vi "UHR-Fleezers Control (host) - 10.6.vi"() -> ()   [LabVIEW 2010] (continued)
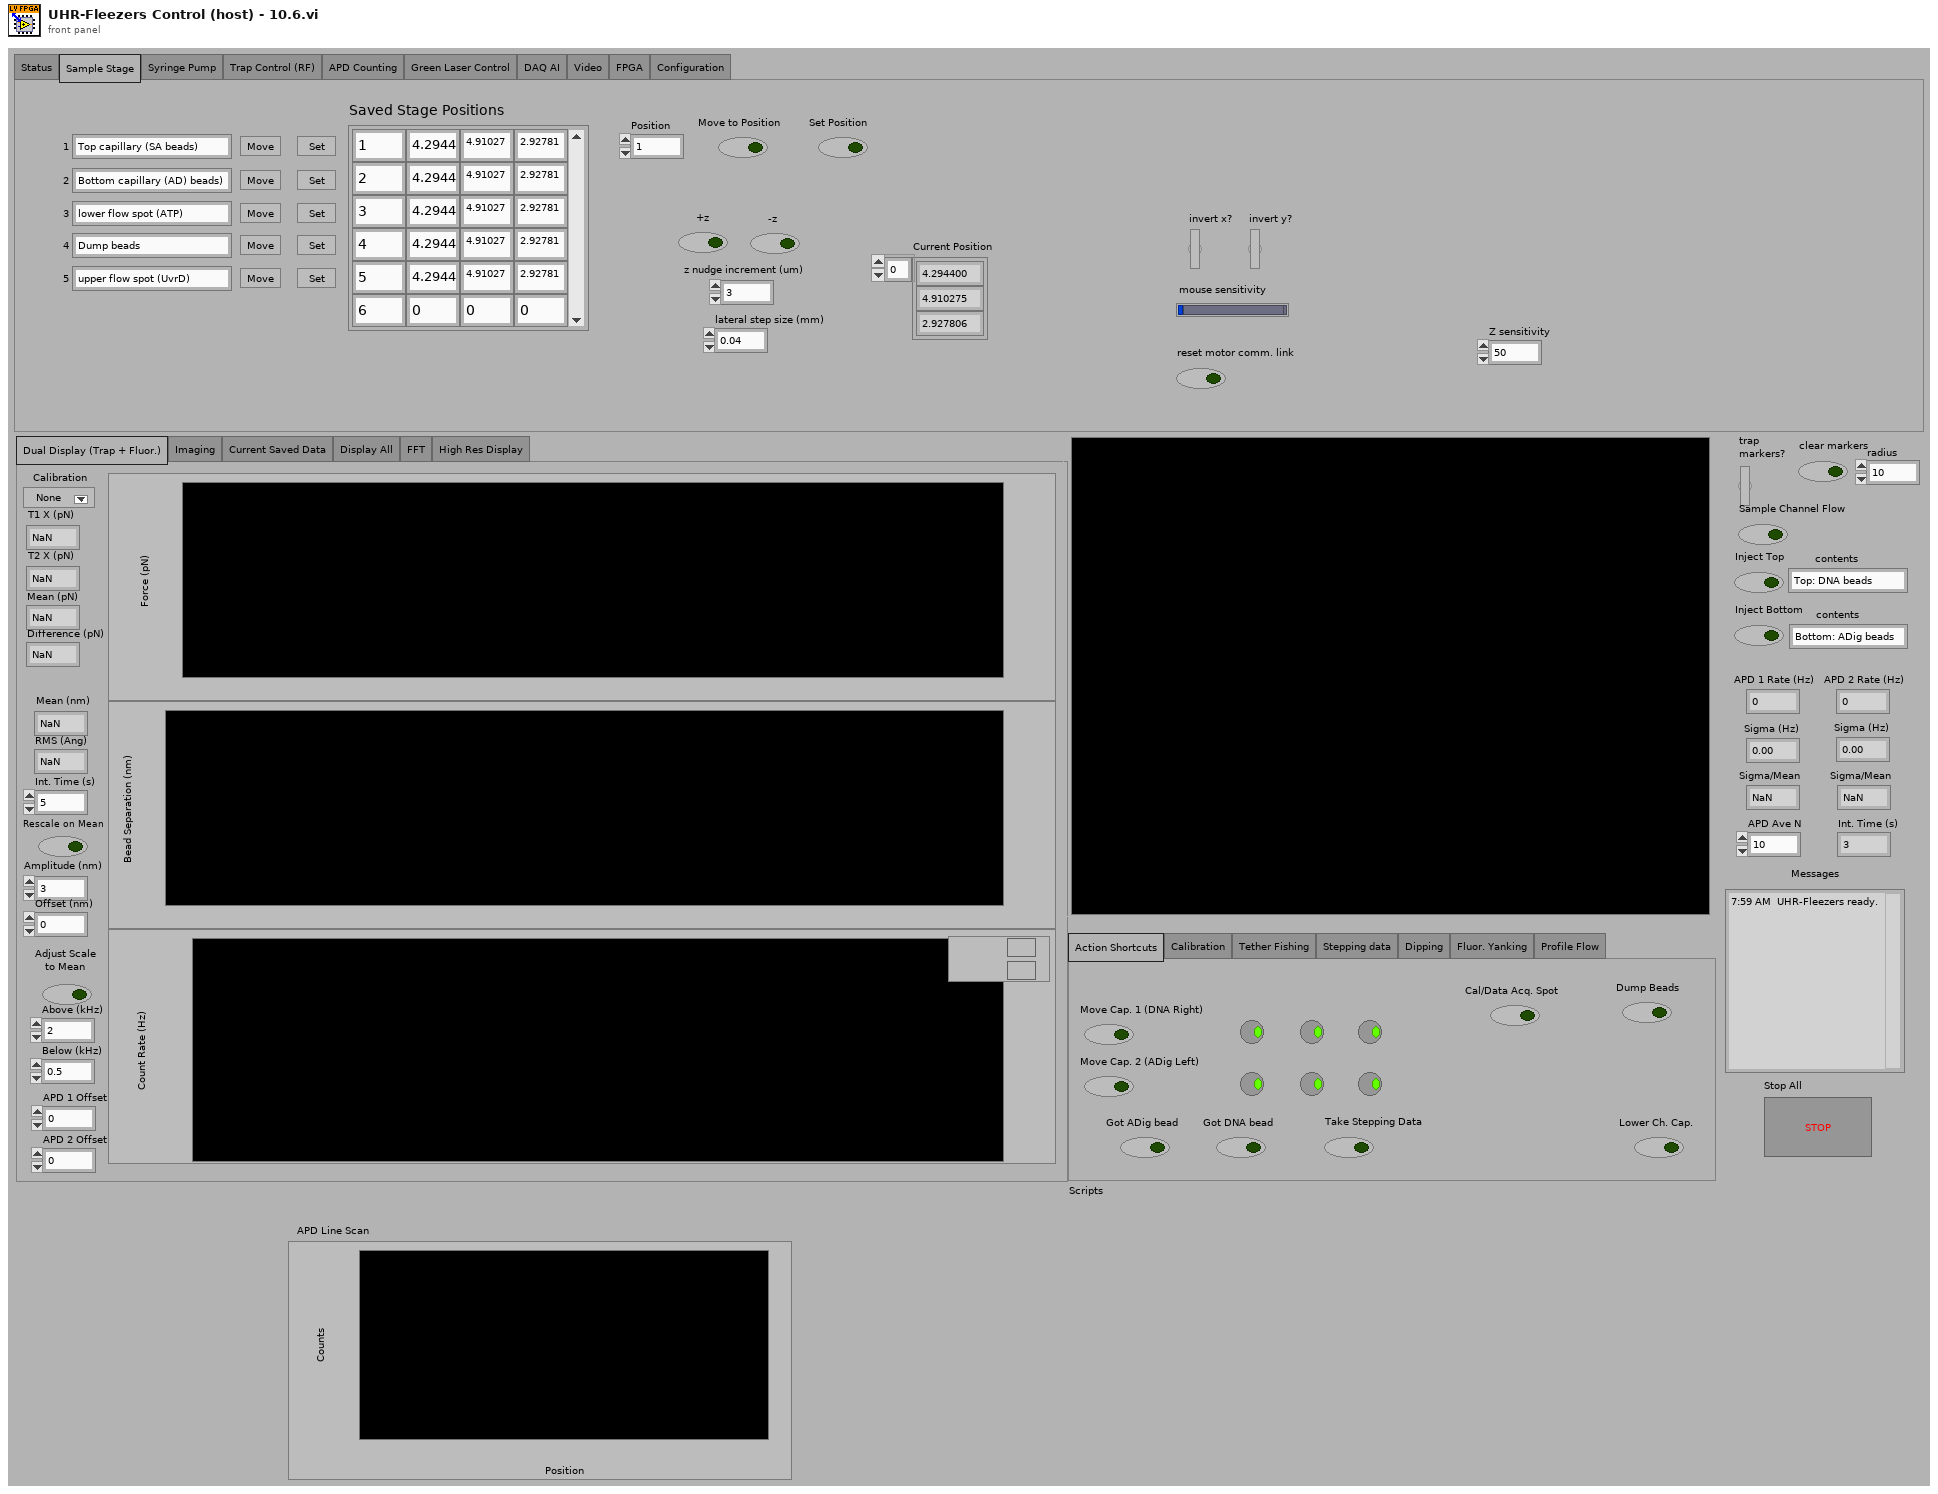
[diagram p1: front panel]
types:
  T1 = enum32{"Action Shortcuts", "Calibration", "Tether Fishing", "Stepping data", "Dipping", "Fluor. Yanking", "Profile Flow"}
  T2 = typedef "IMAQ Image.ctl" = refnum<image>
  T3 = enum32{"Dual Display (Trap + Fluor.)", "Imaging", "Current Saved Data", "Display All", "FFT", "High Res Display"}
  T4 = enum32{"Status", "Sample Stage", "Syringe Pump", "Trap Control (RF)", "APD Counting", "Green Laser Control", "DAQ AI", "Video", "FPGA", "Configuration"}
  T5 = cluster{"Pump 1":cluster{"Diameter (mm)":dbl, "Units":dbl, "Volume":dbl, "Rate":dbl}, "Pump 2":cluster{"Diameter (mm)":dbl, "Units":dbl, "Volume":dbl, "Rate":dbl}, "Pump 3":cluster{"Diameter (mm)":dbl, "Units":dbl, "Volume":dbl, "Rate":dbl}}
  T6 = enum32{"IR Laser Interlacing (Direct RF Board Control Method)", "AOD Raster Scan", "Feedback on Trap Intensity", "Feedback on Trap Position"}
  T7 = typedef "LVPoint32TypeDef.ctl" = cluster{"Horizontal":i32, "Vertical":i32}
  T8 = cluster{"Scan Range AOD (nm) 2":dbl, "Step Size AOD (nm) 2":dbl, "Scan Speed AOD (nm/s) 2":dbl, "Number of scans (AOD) 2":u16, "Label":string}[]
  T9 = cluster{"Set 1":cluster{"proportional gain (Kc)":i16, "integral gain (Kc*Ts/Ti)":i16, "derivative gain (Kc*Td/Ts)":i16}, "Set 2":cluster{"proportional gain (Kc)":i16, "integral gain (Kc*Ts/Ti)":i16, "derivative gain (Kc*Td/Ts)":i16}}
  T10 = cluster{"Trap 1":fxp<+/-,16,1>, "Trap 2":fxp<+/-,16,1>}
  T11 = cluster{"proportional gain (Kc)":fxp<+/-,16,8>, "integral gain (Kc*Ts/Ti)":fxp<+/-,16,8>, "derivative gain (Kc*Td/Ts)":fxp<+/-,16,8>}
  T12 = cluster{"output high":fxp<+/-,16,1>, "output low":fxp<+/-,16,1>}
  T13 = cluster{"Set 1":fxp<+/-,16,1>, "Set 2":fxp<+/-,16,1>}
  T14 = cluster{"proportional gain (Kc)":i16, "integral gain (Kc*Ts/Ti)":i16, "derivative gain (Kc*Td/Ts)":i16}
  T15 = cluster{"Set 1":bool, "Set 2":bool, "Set 3":bool}
  T16 = typedef "LVMinMaxIncTypeDef.ctl" = cluster{"Minimum":dbl, "Maximum":dbl, "Increment":dbl}
  T17 = enum16{"CONNECT", "INITIALIZE VALVES", "DISCONNECT", "MOVE VALVE"}
  T18 = typedef "Image Type" = u32
  T19 = typedef "nirio_resource_hc.ctl" = tag
  T20 = typedef "openfpgaref.8.6.ctl" = refnum<k20>
  T21 = typedef "niFpgaNodeNameForErrorReporting.ctl" = enum16{"Open FPGA VI Reference", "Read/Write Control", "Invoke Method: Abort", "Invoke Method: Acknowledge IRQ", "Invoke Method: Download", "Invoke Method: FIFO.Configure", "Invoke Method: FIFO.Read", "Invoke Method: FIFO.Start", "Invoke Method: FIFO.Stop", "Invoke Method: FIFO.Write", "Invoke Method: Reset", "Invoke Method: Run", "Invoke Method: Wait on IRQ", "Close FPGA VI Reference"}
  T22 = typedef "niLvFpgaWhatHappensToTopLevelVI.ctl" = enum16{"top level VI scripted behind XNode", "top level VI inlined behind XNode"}
  T23 = enum16{"GET STATUS", "ABS MOVE", "GET POS", "REL MOVE", "INIT", "CLOSE", "HOME", "READ ASCII", "ASCII", "SET ULIM", "STOP", "SET LLIM"}
  T24 = cluster{"New Image":T2, "New Image":T2, "New Image":T2, "New Image":T2}
  T25 = enum16{"open", "replace", "create", "open or create", "replace or create", "replace or create with confirmation"}
  T26 = typedef "XDNodeRunTimeDep.lvlib/timing_clust.ctl" = cluster{"Expected End [f-1]":u64, "Actual End [f-1]":u64, "Finished Late? [f-1]":bool, "Expected End [i-1]":u64, "Actual End [i-1]":u64, "Finished Late? [i-1]":bool, "Expected Start [i]":u64, "Actual Start [i]":u64, "Expected Start [f]":u64, "Actual Start [f]":u64, "Source Name":string, "Structure Name":string, "Period":i64, "Deadline":i64, "Offset":i64, "Start":i64, "Priority":i32, "Timeout":i32, "Mode":T27, "Wakeup Reason":T28, "Error":errorcluster, "Source Type":string, "Secondary Source Type":string, "Global End Time":u64, "Global Start Time":u64, "Frame Duration":u64, "Iteration Duration":u64, "Assigned CPU":i32, "I/O Scan Engine Mode":u32}
  T27 = typedef "XDNodeRunTimeDep.lvlib/nitl_modes.ctl" = enum32{"No Change", "Process missed periods, maintain original phase", "Discard missed periods, maintain original phase", "Process missed periods, ignore original phase", "Discard missed periods, ignore original phase"}
  T28 = typedef "XDNodeRunTimeDep.lvlib/wakeup.ctl" = enum32{"Normal", "Aborted", "Asynchronous wakeup", "Timing source error", "Timed loop error", "Timeout"}
  T29 = cluster{"[0]":i32, "[1]":i32, "[2]":i32, "[3]":i32}
  T30 = cluster{"[0]":i32, "[1]":i32, "[2]":i32, "[3]":i32}[]
  T31 = cluster{"Horizontal":i32, "Vertical":i32, "Scrolling":i32}
  T32 = enum32{"Normal Display", "Dual Display (APD)", "FFT", "High Res Display"}
  T33 = cluster{"Origin Pixel":cluster{"X":sgl, "Y":sgl}, "Angle Relative to Horizontal (deg)":sgl, "Axis Reference":u32}
  T34 = typedef "Simple Grid Descriptor" = cluster{"X Step":sgl, "Y Step":sgl, "Unit":T35}
  T35 = typedef "Image Unit" = enum32{"Undefined", "Angström", "Micrometer", "Millimeter", "Centimeter", "Meter", "Kilometer", "Microinch", "Inch", "Feet", "Nautical miles", "Standard miles", "Steps"}
  T36 = cluster{"averaging mode":u16, "weighting mode":u16, "number of averages":u32}
  T37 = cluster{"dB On (F)":bool, "unwrap phase (F)":bool, "convert to degree (F)":bool}
  T38 = cluster{"Green FB Ch 0":i16, "Green FB Ch 1":i16, "Green FB Ch 2":i16}
  T39 = enum16{"big-endian, network order", "native, host order", "little-endian"}
  T40 = cluster{string, string, string, string, string, string, string, string}
  T41 = cluster{string, string, string, string, string, string, string, string, string, string, string, string}
  T42 = cluster{string, string, string, string, string, string, string, string, string, string, string, string, string}
  T43 = cluster{string, string, string, string, string, string, string, string, string, string, string, string, string, string}
  T44 = cluster{"BD 1 Frequency 1 (MHz)":dbl, "BD 1 Frequency 2 (MHz)":dbl}
  T45 = cluster{"f0":dbl, "df":dbl, "magnitude":dbl[]}[][]
  T46 = cluster{"Green FB Ch 0":dbl, "Green FB Ch 1":dbl, "Green FB Ch 2":dbl}
  T47 = enum16{"Always On", "Always Off", "Off While Running"}
  T48 = cluster{"Scan Range AOD (nm) 2":dbl, "Step Size AOD (nm) 2":dbl, "Scan Speed AOD (nm/s) 2":dbl, "Number of scans (AOD) 2":u16, "Label":string}
  T49 = typedef "eventvkey.ctl" = enum16{"ASCII", "Enter", "Return", "Shift", "Ctrl", "Alt", "Cmd", "Opt", "Caps", "NumLock", "Clear", "Break", "Up", "Down", "Left", "Right", "Insert", "Delete", "Home", "End", "PageUp", "PageDown", "Escape", "Help", "Pause", "ScrollLock", "F1", "F2", "F3", "F4", "F5", "F6", "F7", "F8", "F9", "F10", "F11", "F12", "F13", "F14", "F15", "F16", "F17", "F18", "F19", "F20", "F21", "F22", "F23", "F24", "Play", "VolumeUp", "VolumeDown", "Mute", "Two Byte Char"}
  T50 = cluster{"[0]":dbl, "[1]":dbl, "[2]":dbl, "[3]":dbl, "[4]":dbl, "[5]":dbl}
  T51 = cluster{"Diameter (mm)":dbl, "Units":dbl, "Volume":dbl, "Rate":dbl}
  T52 = cluster{"Left":i32, "Top":i32, "Width":u32, "Height":u32}
  T53 = cluster{cluster{"Left":i32, "Top":i32, "Width":u32, "Height":u32}}[]
diagram:
  w62 = u16 20 items=["1.0"=10, "1.5"=15, "2.0"=20] ("stop bits (10: 1 bit)")
  w69 = T18 2 items=["Grayscale (U8)", "Grayscale (I16)", "Grayscale (SGL)", "Complex (CSG)", "RGB (U32)", "HSL (U32)", "RGB (U64)", "Grayscale (U16)"] ("Image Type")
  w126 = cluster{"output high":i16, "output low":i16} {"output high"=3000, "output low"=0} ("FB output range 1")
  w201 = 10.0 ("y")
  w200 = 32767.0 ("y")
  w216 = 6.0  # clock mult.
  w217 = 49152000.0  # TCXO frequ.
  n1 = Build Array("DIO count 1 (ticks)", "DIO count 2 (ticks)", "DIO count 3 (ticks)") -> (w115:u32[])
  n2 = Multiply(x="APD Integration Time (s)", y=40000000.0) -> (x*y=w133:dbl)
  n3 = Reciprocal(x="APD Integration Time (s)") -> (1/x=w130:dbl)
  n4 = local write "APD Acq Rate (Hz)"(w130) -> ()
  n5 = local read "AO1"() -> (w195:dbl)
  n6 = local read "AO2"() -> (w194:dbl)
  n7 = To Unsigned Long Integer(number=w133) -> (unsigned 32bit integer=w132:u32)
  "APD Int. Count" <- w132
  n8 = local read "Scan Increment (MHz)"() -> (w212:dbl)
  n9 = local read "Continuous MCL Scanning"() -> (w182:bool)
  n10 = local read "Fast Scan Dir"() -> (w181:bool)
  n11 = local read "Trap Intensity\nSetpoints (V)"() -> (w231:cluster{"Set 1":dbl, "Set 2":dbl})
  n12 = local read "Number of scans (MCL)"() -> (w183:u64)
  n13 = Multiply(x=w195, y=w200) -> (x*y=w197:dbl)
  n14 = Multiply(x=w194, y=w200) -> (x*y=w199:dbl)
  n15 = Divide(x=w197, y=w201) -> (x/y=w196:dbl)
  n16 = Divide(x=w199, y=w201) -> (x/y=w198:dbl)
  n17 = To Word Integer(number=w196) -> (16bit integer=w193:i16)
  n18 = To Word Integer(number=w198) -> (16bit integer=w192:i16)
  n19 = Not(x=w181) -> (.not. x?=w176:bool)
  n20 = local read "Cycles/step (MCL)"() -> (w184:u64)
  n21 = Multiply(x=w212, y=1000.0) -> (x*y=w219:dbl)
  n22 = local read "Scan steps (MCL)"() -> (w185:u64)
  n23 = local write "Trap Pos FIFO Timeout"(u16 0 ("Trap Pos FIFO Timeout")) -> ()
  n24 = local read "Desired Scan Incr (V)"() -> (w187:dbl)
  n25 = Scale By Power Of 2(n=48, x=w219) -> (x*2^n=w220:dbl)
  n26 = Multiply(x=w217, y=w216) -> (x*y=w215:dbl)
  n27 = Divide(x=w220, y=w215) -> (x/y=w214:dbl)
  n28 = local read "Number Interlace Sets"() -> (w108:u8)
  n29 = Split 1D Array(array=w115, index=w108) -> (first subarray=w117:u32[])  [unwired: 1 out]
  n30 = Add Array Elements(numeric array=w117) -> (sum=w116:u32)
  n31 = property on="AI Count (ticks)" class="DigNum (strict)"("Val(Sgnl)"="AI Count (ticks)") -> ()  [unwired: 2 in, 2 out]
  n32 = local read "# Samples/channel"() -> (w204:u32)
  n33 = local read "Number of F/B Scans (AOD)"() -> (w205:u16)
  n34 = To Quad Integer(1:w214) -> (0:w211:i64)
  n35 = local read "Not-Interlacing Set"() -> (w107:enum32{"Set 1", "Set 2", "Set 3"})
  n36 = To Unsigned Byte Integer(number=w107) -> (unsigned 8bit integer=w113:u8)
  n37 = Index Array(array=w115, index=w113) -> (element=w114:u32)
  n38 = local read "Feedback On/Off"() -> (w234:cluster{"Set 1":bool, "Set 2":bool})
  n39 = local read "PID Gains"() -> (w226:T9)
  n40 = Divide(x=40000000.0, y="AI Count (ticks)") -> (x/y=w173:dbl)
  n41 = Multiply(x=w187, y=32767.0) -> (x*y=w189:dbl)
  n42 = local read "Scan steps (AOD)"() -> (w210:u64)
  n43 = local read "All FB On/Off"() -> (w235:bool)
  n44 = local read "Cycles/step (AOD)"() -> (w209:u64)
  n45 = local write "AI rate (Hz)"(w173) -> ()
  n46 = Divide(x=w189, y=10.0) -> (x/y=w188:dbl)
  n47 = Multiply(x=w210, y=w209) -> (x*y=w208:u64)
  n48 = Multiply(x=3276.7, y=w231) -> (x*y=w230:cluster{"Set 1":dbl, "Set 2":dbl})
  n49 = To Word Integer(number=w188) -> (16bit integer=w186:i16)
  n50 = Multiply(x=w208, y=u64 2) -> (x*y=w206:u64)
  n51 = local read "Sets to FIFO (Traps)"() -> (w238:T15)
  n52 = Divide(x=w173, y="FPGA Ave.") -> (x/y=w174:dbl)
  n53 = To Word Integer(number=w230) -> (16bit integer=w229:cluster{"Set 1":i16, "Set 2":i16})
  n54 = xnode "Open FPGA VI Reference"("resource name"=T19 "750kHzDAQ") -> ("FPGA VI Reference Out"=w223:T20)  [unwired: 1 in, 1 out]
  n55 = Unbundle By Name(w226) -> ("Set 1"=w225:T14, "Set 2"=w224:T14)
  n56 = Multiply(x=w206, y=w205) -> (x*y=w203:u64)
  n57 = local write "Ave. Rate (Hz)"(w174) -> ()
  n58 = Divide(x=w203, y=w204) -> (x/y=w202:dbl)
  n59 = Unbundle By Name(w229) -> ("Set 1"=w228:i16, "Set 2"=w227:i16)
  n60 = local read "2D or 1D Scan"() -> (w127:bool)
  n61 = local write "Data points/scans"(w203) -> ()
  n62 = local read "Scan BD"() -> (w221:bool)
  n63 = And(x=w234, y=w235) -> (x .and. y?=w233:cluster{"Set 1":bool, "Set 2":bool})
  n64 = local write "Data points/scan (f/b)"(w206) -> ()
  n65 = Reciprocal(x=w174) -> (1/x=w175:dbl)
  n66 = local read "N Acq Sets (Traps + Fl.)"() -> (w166:i16)
  n67 = local write "N sets should be saved"(w202) -> ()
  n68 = Unbundle By Name(w233) -> ("Set 1"=w237:bool, "Set 2"=w236:bool)
  n69 = local read "Interlace"() -> (w109:bool)
  n70 = Select(t=w116, s=w109, f=w114) -> (s? t:f=w106:u32)
  n71 = local write "Update Count (MCL)"(w106) -> ()
  n72 = local write "Total Counts (ticks)"(w106) -> ()
  n73 = xnode "Invoke Method"("FPGA VI Reference In"=w223) -> ("FPGA VI Reference Out"=w125:T20, "error out"=w144:errorcluster)  [unwired: 1 in]
  n74 = local write "Ave. Period (s)"(w175) -> ()
  n75 = property on="2D or 1D Scan" class="Bool (strict)"("Val(Sgnl)"=w127) -> ()  [unwired: 2 in, 2 out]
  n76 = xnode "Read/Write Control"("FPGA VI Reference In"=w124, "error in"=w144, "ai count"="AI Count (ticks)", "Interlace ON/OFF"=w109, "Number Interlace Cycles"=w108, "AI1 Sets to FIFO"=w238, "FB On/Off Set 1"=w237, "FB On/Off Set 2"=w236, "Interlace Off Parameters"=w107, "FB Setpoint Set 1"=w228, "FB Setpoint Set 2"=w227, "FB Gains Set 1"=w225, "FB Gains Set 2"=w224, "FB output range 1"=w126, "FB output range 2"=w126, "Cycles per step"=w209, "Scan BD"=w221, "Number of scans"=w205, "Scan steps"=w210, "Scan freq.  increment"=w211, "AO1"=w193, "AO2"=w192, "Scan freq.  increment (MCL)"=w186, "Scan steps (MCL)"=w185, "Cycles per step (MCL)"=w184, "Number of scans (MCL)"=w183, "MCL count"=w106, "Cont. Scan (MCL)"=w182, "MCL Scan Axis"=w176, "1D or 2D Scan?"=w127, "N of AI1 Int Acq Sets"=w166, "Freq or Amp switch first"="Freq or Amp switch first", "Freq switch delay"="Freq switch delay", "Amp switch delay"="Amp switch delay", "Swap F1 and F2"="Swap F1 and F2", "APD Acq Rate Count"=w132, "APD to FIFO"=FALSE, "APD Gate Operating Mode"="APD Gate", "APD Gate ON Count"="APD Gate ON Count", "APD Gate OFF Count"="APD Gate OFF Count", "Invert APD Gate"="Invert APD Gate", "DIO count 1 (ticks)"="DIO count 1 (ticks)", "DIO count 2 (ticks)"="DIO count 2 (ticks)", "DIO count 3 (ticks)"="DIO count 3 (ticks)", "APD 1 AO scale factor"="APD 1 AO Mult.", "APD 2 AO scale factor"="APD 2 AO Mult.") -> ("FPGA VI Reference Out"=w101:T20, "error out"=w103:errorcluster)  [unwired: 1 in]
  n77 = local read "Green Laser ON/Interlacing"() -> (w104:bool)
  n78 = local read "Green laser mode"() -> (w105:enum32{"Laser ON", "Laser OFF", "Interlace"})
  n79 = local read "GI Frequency, OFF count"() -> (w97:u32)
  n80 = local read "GI Frequency, ON count"() -> (w96:u32)
  n81 = Multiply(x="Current When FB OFF (%)", y=655.35) -> (x*y=w87:dbl)
  n82 = local read "Green FB Count"() -> (w95:u32)
  n83 = Multiply(x="Green FB Setpoint (mV)", y=3.2767) -> (x*y=w84:dbl)
  n84 = To Unsigned Word Integer(number=w87) -> (unsigned 16bit integer=w85:u16)
  n85 = local read "Invert GI"() -> (w99:bool)
  n86 = To Word Integer(number=w84) -> (16bit integer=w82:i16)
  n87 = case shown="True" w104 {
    tunnel: w105 -> [_ w258]
    tunnel: [enum32{"Laser ON", "Laser OFF", "Interlace"}."Laser OFF" ("Green laser mode") w258] -> w98
    frame False {
    }
    frame True {
    }
  }
  n88 = local read "Trap Pos. AI1 X Pre-scale"() -> (w49:u16)
  n89 = local read "Trap Pos FB Monitor\nT1 or T2"() -> (w56:bool)
  n90 = local read "Trap Pos FB Int Count"() -> (w44:u16)
  n91 = local read "Trap Pos FB Negate Action"() -> (w55:bool)
  n92 = local read "Trap Pos. FB Offset Factor"() -> (w54:i64)
  n93 = local read "Trap Pos. FB Mult Factor"() -> (w53:i64)
  n94 = local read "Trap Pos. FB Gains"() -> (w51:T11)
  n95 = local read "Trap Pos. FB Range"() -> (w52:T12)
  n96 = xnode "Read/Write Control"("FPGA VI Reference In"=w101, "error in"=w103, "Green interlace ON count 2"=w96, "Green interlace OFF count 2"=w97, "Invert GI 2"=w99, "Operating Mode 2"=w98, "Green FB Gains"="Green FB Gains", "Green FB Setpoint"=w82, "Green FB On/Off"="Green FB On/Off", "Current Out"=w85, "Green int current ON count adj"="Green int current ON count adj", "Green FB Count"=w95, "Operating Mode"=w98, "Green interlace OFF count"=w97, "Green interlace ON count"=w96, "Invert GI"=w99, "Trap Pos FB Monitor T1 or T2"=w56, "Trap Pos FB Negate Action"=w55, "Trap Pos. FB Offset Factor"=w54, "Trap Pos. FB Mult Factor"=w53, "Trap Pos. FB Range"=w52, "Trap Pos. FB Gains"=w51, "Force feedback"=FALSE, "AI1 X Scale"=w49, "Trap Pos to FIFO"=TRUE, "Trap Pos FB Int Count"=w44) -> ("FPGA VI Reference Out"=w100:T20, "error out"=w102:errorcluster)
  n97 = xnode "Invoke Method"("FPGA VI Reference In"=w100, "error in"=w102, "Depth"="Trap AI FIFO Depth") -> ("FPGA VI Reference Out"=w59:T20, "error out"=w58:errorcluster)
  n98 = xnode "Invoke Method"("FPGA VI Reference In"=w59, "error in"=w58, "Depth"="Trap Position FIFO Depth") -> ("FPGA VI Reference Out"=w46:T20, "error out"=w45:errorcluster)
  n99 = flat-sequence {
    tunnel: w125 -> [w263]
    tunnel: [w263] -> w124
    tunnel: [w262] -> w123
    tunnel: [w261] -> w122
    tunnel: [w259] -> w120
    tunnel: [w260] -> w121
    frame #0 {
      w260 = T16 {"Minimum"=50.0, "Maximum"=100.0, "Increment"=1.0} ("Min Max Inc")
      w259 = T16 {"Minimum"=0.0, "Maximum"=75.0, "Increment"=1.0} ("Data Entry Limits")
      w262 = T16 {"Minimum"=50.0, "Maximum"=100.0, "Increment"=1.0} ("Min Max Inc")
      w261 = T16 {"Minimum"=0.0, "Maximum"=75.0, "Increment"=1.0} ("Data Entry Limits")
      n100 = property on="BD 2 Frequency 1 (MHz)" class="DigNum (strict)"("Data Range"=w260) -> ()  [unwired: 2 in, 2 out]
      n101 = property on="BD 2 Frequency 3 (MHz)" class="DigNum (strict)"("Data Range"=w260) -> ()  [unwired: 2 in, 2 out]
      n102 = property on="BD 2 Frequency 2 (MHz)" class="DigNum (strict)"("Data Range"=w260) -> ()  [unwired: 2 in, 2 out]
      n103 = property on="BD 1 Frequency 1 (MHz)" class="DigNum (strict)"("Data Range"=w262) -> ()  [unwired: 2 in, 2 out]
      n104 = property on="BD 1 Frequency 2 (MHz)" class="DigNum (strict)"("Data Range"=w262) -> ()  [unwired: 2 in, 2 out]
      n105 = property on="BD 1 Frequency 3 (MHz)" class="DigNum (strict)"("Data Range"=w262) -> ()  [unwired: 2 in, 2 out]
      n106 = property on="BD 2 Amplitude 1 (%)" class="DigNum (strict)"("Data Range"=w259) -> ()  [unwired: 2 in, 2 out]
      n107 = property on="BD 2 Amplitude 2 (%)" class="DigNum (strict)"("Data Range"=w259) -> ()  [unwired: 2 in, 2 out]
      n108 = property on="BD 2 Amplitude 3 (%)" class="DigNum (strict)"("Data Range"=w259) -> ()  [unwired: 2 in, 2 out]
      n109 = property on="BD 1 Amplitude 3 (%)" class="DigNum (strict)"("Data Range"=w261) -> ()  [unwired: 2 in, 2 out]
      n110 = property on="BD 1 Amplitude 2 (%)" class="DigNum (strict)"("Data Range"=w261) -> ()  [unwired: 2 in, 2 out]
      n111 = property on="BD 1 Amplitude 1 (%)" class="DigNum (strict)"("Data Range"=w261) -> ()  [unwired: 2 in, 2 out]
      "X RF Frequency Limits (MHz)" <- w262
      "X RF Amplitude Limits (%)" <- w261
      "Y RF Amplitude Limits (%)" <- w259
      "Y RF Frequency Limits (MHz)" <- w260
    }
  }
  n112 = xnode "Invoke Method"("FPGA VI Reference In"=w46, "error in"=w45) -> ("FPGA VI Reference Out"=w16:T20, "error out"=w15:errorcluster)  [unwired: 1 out]
  n113 = flat-sequence "Initial FPGA Loop Relative Phase Adjustment" {
    tunnel: "Initial Phase Adjustment (APD 2 Gate)" -> [w265]
    tunnel: "Initial Phase Adjustment (GI) 2" -> [w266]
    tunnel: "Initial Phase Adj. (MCL)" -> [w267]
    tunnel: w15 -> [w268]
    tunnel: w16 -> [w269]
    tunnel: "Initial Phase Adjustment (GI)" -> [w270]
    tunnel: "Initial Phase Adjustment (AI1)" -> [w271]
    tunnel: [w271] -> w30
    tunnel: [w270] -> w29
    tunnel: [w269] -> w28
    tunnel: [w268] -> w27
    tunnel: [w267] -> w26
    tunnel: [w266] -> w25
    tunnel: [w265] -> w24
    tunnel: [w283] -> w150
    tunnel: [w277] -> w148
    tunnel: "Initial Phase Adjustment (APD Acq)" -> [w276]
    tunnel: "Initial Phase Adjustment (APD 1 Gate)" -> [w275]
    tunnel: "Initial Phase Adjustment (Green FB)" -> [w274]
    tunnel: w30 -> [w282]
    tunnel: w29 -> [w281]
    tunnel: w28 -> [w280]
    tunnel: w27 -> [w279]
    tunnel: w26 -> [w278]
    tunnel: w25 -> [w273]
    tunnel: w24 -> [w272]
    tunnel: w150 -> [w462]
    tunnel: [w463] -> w149
    tunnel: w148 -> [w463]
    tunnel: [w462] -> w147
    tunnel: w149 -> [w466]
    tunnel: w147 -> [w465]
    tunnel: [w468] -> w146
    tunnel: [w467] -> w145
    tunnel: [w655] -> w14
    tunnel: [w656] -> w17
    tunnel: w146 -> [w656]
    tunnel: w145 -> [w655]
    frame #0 {
      n114 = Wait (ms)(milliseconds to wait=u32 1000) -> ()  [unwired: 1 out]
    }
    frame #1 {
      n115 = xnode "Read/Write Control"("FPGA VI Reference In"=w280, "error in"=w279, "Phase count adjustment"=w282, "Phase count adjustment (GI)"=w281, "Phase count adjustment (MCL)"=w278, "Phase Count Adjustment (APD Acq)"=w276, "Phase count adjustment (APD 1 Gate)"=w275, "Phase count adjustment (APD 2 Gate)"=w272, "Phase count adjustment (Green FB)"=w274, "Phase count adjustment (GI) 2"=w273) -> ("FPGA VI Reference Out"=w277:T20, "error out"=w283:errorcluster)
    }
    frame #2 {
      n116 = Wait (ms)(milliseconds to wait=u32 1000) -> ()  [unwired: 1 out]
    }
    frame #3 {
      w464 = TRUE
      n117 = xnode "Read/Write Control"("FPGA VI Reference In"=w466, "error in"=w465, "+ phase"=w464, "+ phase (GI)"=w464, "+ phase (MCL)"=w464, "+ phase (APD Acq)"=w464, "+ phase (APD 1 Gate)"=w464, "+ phase (APD 2 Gate)"=w464, "+ phase (Green FB)"=w464, "+ phase (GI) 2"=w464) -> ("FPGA VI Reference Out"=w467:T20, "error out"=w468:errorcluster)
    }
    frame #4 {
      n118 = Wait (ms)(milliseconds to wait=u32 1000) -> ()  [unwired: 1 out]
    }
  }
  n119 = local read "Phase adj. (Green FB)"() -> (w118:i16)
  n120 = local read "Phase adj. (GI) 2"() -> (w88:i16)
  n121 = local read "Phase adjust (MCL)"() -> (w177:i16)
  n122 = local read "Phase adj. (AI1)"() -> (w179:i16)
  n123 = local read "Phase adj. (GI)"() -> (w178:i16)
  n124 = xnode "Read/Write Control"("FPGA VI Reference In"=w14, "error in"=w17, "Phase count adjustment"=w179, "Phase count adjustment (GI)"=w178, "Phase count adjustment (MCL)"=w177, "Phase Count Adjustment (APD Acq)"="Phase Adj. (APD Acq)", "Phase count adjustment (APD 1 Gate)"="Phase Adj. (APD 1 Gate)", "Phase count adjustment (APD 2 Gate)"="Phase Adj. (APD 2 Gate)", "Phase count adjustment (Green FB)"=w118, "Phase count adjustment (GI) 2"=w88) -> ("FPGA VI Reference Out"=w13:T20, "error out"=w12:errorcluster)
  n125 = call "Initialize RF boards - interlace 3.vi"("error in"=w12, "FPGA VI Reference In"=w13) -> ("FPGA VI Reference Out"=w155:T20)  [unwired: 1 out]
  n126 = call "set RF board frequency - interlace.vi"("Board 2 Frequency Limits"=w121, "Board 1 Frequency Limits"=w123, "FPGA VI Reference In"=w155, "Board 2 Frequency 3 (MHz)"="BD 2 Frequency 3 (MHz)", "Board 1 Frequency 3 (MHz)"="BD 1 Frequency 3 (MHz)", "Board 2 Frequency 2 (MHz)"="BD 2 Frequency 2 (MHz)", "Board 2 Frequency 1 (MHz)"="BD 2 Frequency 1 (MHz)", "Board 1 Frequency 2 (MHz)"="BD 1 Frequency 2 (MHz)", "Board 1 Frequency 1  (MHz)"="BD 1 Frequency 1 (MHz)") -> ("error out"=w249:errorcluster, "FPGA VI Reference Out"=w250:T20)  [unwired: 1 in]
  n127 = call "set RF board amplitude - interlace.vi"("Board 2 Amplitude Limits"=w120, "Board 1 Amplitude Limits"=w122, "error in"=w249, "FPGA VI Reference In"=w250, "Board 2 Amplitude 3 (%)"="BD 2 Amplitude 3 (%)", "Board 1 Amplitude 3 (%)"="BD 1 Amplitude 3 (%)", "Board 2 Amplitude 2 (%)"="BD 2 Amplitude 2 (%)", "Board 2 Amplitude 1 (%)"="BD 2 Amplitude 1 (%)", "Board 1 Amplitude 2 (%)"="BD 1 Amplitude 2 (%)", "Board 1 Amplitude 1 (%)"="BD 1 Amplitude 1 (%)") -> ("error out"=w10:errorcluster, "FPGA VI Reference Out"=w11:T20)
  n128 = flat-sequence {
    tunnel: w11 -> [w665]
    tunnel: w10 -> [w664]
    tunnel: [w663] -> w242
    tunnel: [w662] -> w241
    tunnel: [w707] -> w240
    tunnel: w242 -> [w707]
    tunnel: [w706] -> w239
    tunnel: w241 -> [w706]
    tunnel: w240 -> [w716]
    tunnel: w239 -> [w715]
    tunnel: [w714] -> w40
    tunnel: [w713] -> w39
    tunnel: w40 -> [w781]
    tunnel: w39 -> [w776]
    tunnel: [w781] -> w4
    tunnel: [w772] -> w3
    tunnel: [w784] -> w41
    tunnel: [w789] -> w18
    tunnel: w4 -> [w789]
    tunnel: w3 -> [w785]
    frame #0 {
      n129 = local read "Trap 1 (ON/OFF)"() -> (w657:bool)
      n130 = xnode "Read/Write Control"("FPGA VI Reference In"=w665, "error in"=w664, "Direct RF Box  Communication"=FALSE) -> ("FPGA VI Reference Out"=w663:T20, "error out"=w662:errorcluster)
      n131 = local write "Saving..."(FALSE ("Saving Data")) -> ()
      n132 = local write "Stop All"(FALSE ("Stop All")) -> ()
      n133 = local write "Index"(1.0 ("Index")) -> ()
      n134 = property on="Trap 1 ON" class="Bool (strict)"("Value"=w657) -> ()  [unwired: 2 in, 2 out]
      "Manipulating Trap" <- FALSE ("Manipulating Trap")
    }
    frame #1 {
      n135 = local read "Trap 2 (ON/OFF)"() -> (w705:bool)
      n136 = Wait (ms)(milliseconds to wait=u32 50) -> ()  [unwired: 1 out]
      n137 = property on="Trap 2 ON" class="Bool (strict)"("Val(Sgnl)"=w705) -> ()  [unwired: 2 in, 2 out]
    }
    frame #2 {
      n138 = local read "Scan Range (nm)"() -> (w709:dbl)
      n139 = xnode "Read/Write Control"("FPGA VI Reference In"=w716, "error in"=w715, "FPGA Controls  RF Box"=TRUE ("Direct RF Box  Communication")) -> ("FPGA VI Reference Out"=w714:T20, "error out"=w713:errorcluster)
      n140 = call "Update messages.vi"("Message to add"="UHR-Fleezers ready.", "Old message string"="") -> ("New message string"=w712:string)
      n141 = local write "Messages"(w712) -> ()
      n142 = property on="Scan Range (nm)" class="DigNum (strict)"("Val(Sgnl)"=w709) -> ()  [unwired: 2 in, 2 out]
    }
    frame #3 {
      w761 = T23."ASCII" ("Command")
      # "disable hysteresis\ncompensation for\nfaster performance"
      # "increase jerk\nfor faster \nresponse"
      # "disable backlash\ncompensation for\nfaster response \ntimes. necessary\nfor mouse control\nof stage"
      n143 = call "CONEX_FUNCTIONAL_GLOBAL.vi"("error in"=w776, "Command"=T23."INIT") -> ("error out"=w757:errorcluster)  [unwired: 7 in, 2 out]
      n144 = call "CONEX_FUNCTIONAL_GLOBAL.vi"("error in"=w757, "Position"=dbl[] [10.0, 12.0, 2.0], "Command"=T23."SET ULIM") -> ("error out"=w777:errorcluster)  [unwired: 6 in, 2 out]
      n145 = call "CONEX_FUNCTIONAL_GLOBAL.vi"("error in"=w777, "Position"=dbl[] [0.0, 0.0, 4.0], "Command"=T23."SET LLIM") -> ("error out"=w770:errorcluster)  [unwired: 6 in, 2 out]
      n146 = Concatenate Strings("1BA0", "\r\n") -> (w767:string)
      n147 = call "CONEX_FUNCTIONAL_GLOBAL.vi"("error in"=w770, "ASCII command"=w767, "Command"=w761) -> ("error out"=w766:errorcluster)  [unwired: 6 in, 2 out]
      n148 = Concatenate Strings("1JR0.001", "\r\n") -> (w763:string)
      n149 = call "CONEX_FUNCTIONAL_GLOBAL.vi"("error in"=w766, "ASCII command"=w763, "Command"=w761) -> ("error out"=w762:errorcluster)  [unwired: 6 in, 2 out]
      n150 = Concatenate Strings("1BH0", "\r\n") -> (w758:string)
      n151 = call "CONEX_FUNCTIONAL_GLOBAL.vi"("error in"=w762, "ASCII command"=w758, "Command"=w761) -> ("error out"=w756:errorcluster)  [unwired: 6 in, 2 out]
      n152 = call "CONEX_FUNCTIONAL_GLOBAL.vi"("error in"=w756, "Command"=T23."GET POS") -> ("error out"=w772:errorcluster, "Current Position"=w771:dbl[])  [unwired: 7 in, 1 out]
      n153 = local write "Current Position"(w771) -> ()
    }
    frame #4 {
      n154 = call "hamilton_controller.vi"("error in"=w785, "valve"=enum16{"A", "B", "C", "D", "ALL"}."ALL", "action"=T17."CONNECT") -> ("error out"=w786:errorcluster)  [unwired: 8 in]
      n155 = call "hamilton_controller.vi"("error in"=w786, "valve"=enum16{"A", "B", "C", "D", "ALL"}."ALL", "action"=T17."INITIALIZE VALVES") -> ("error out"=w784:errorcluster)  [unwired: 8 in]
    }
  }
  n156 = Subtract(x="BD 1 Frequency 1 (MHz)", y="BD 1 Frequency 2 (MHz)") -> (x-y=w165:dbl)
  n157 = Subtract(x="BD 2 Frequency 1 (MHz)", y="BD 2 Frequency 2 (MHz)") -> (x-y=w164:dbl)
  n158 = Square(x=w164) -> (x^2=w162:dbl)
  n159 = Square(x=w165) -> (x^2=w163:dbl)
  n160 = Add(x=w163, y=w162) -> (x+y=w161:dbl)
  n161 = Square Root(x=w161) -> (sqrt(x)=w160:dbl)
  n162 = local write "Trap Delta (MHz)"(w160) -> ()
  n163 = call "IMAQ Create"("Image Name"="APD 1 Image", "Image Type"=w69) -> ("New Image"=w68:T2)  [unwired: 3 in, 1 out]
  n164 = call "IMAQ Create"("Image Name"="APD 2 Image", "Image Type"=w69) -> ("New Image"=w67:T2)  [unwired: 3 in, 1 out]
  n165 = call "IMAQ Create"("Image Name"="Det. X Image", "Image Type"=w69) -> ("New Image"=w66:T2)  [unwired: 3 in, 1 out]
  n166 = call "IMAQ Create"("Image Name"="Det. Y Image", "Image Type"=w69) -> ("New Image"=w65:T2)  [unwired: 3 in, 1 out]
  n167 = call-poly "VISA Configure Serial Port"("VISA resource name"="Harvard Syringe Pump Serial Port", "baud rate (9600)"=u32 115200, "stop bits (10: 1 bit)"=w62) -> ("VISA resource name out"=w60:refnum<visa-resource-name>)  [unwired: 4 in, 8 out]
  n168 = Bundle("New Image"=w68, "New Image"=w67, "New Image"=w66, "New Image"=w65) -> (w64:T24)  [unwired: 1 in]
  n169 = disable-structure shown="Disabled" {
    disable-tunnel: w18 -> [w804 _]
    frame Disabled {
      w813 = T18 0 items=["Grayscale (U8)", "Grayscale (I16)", "Grayscale (SGL)", "Complex (CSG)", "RGB (U32)", "HSL (U32)", "RGB (U64)", "Grayscale (U16)"] ("Image Type")
      n170 = call <vilib>:"IMAQ Init.vi"("Interface Name"="img0") -> ("error out"=w815:errorcluster, "IMAQ Session Out"=w817:refnum<k11>)  [unwired: 9 in]
      n171 = call <vilib>:"IMAQ Grab Setup.vi"("error in (no error)"=w815, "IMAQ Session In"=w817) -> ("error out"=w811:errorcluster, "IMAQ Session Out"=w812:refnum<k11>)  [unwired: 8 in]
      n172 = call "IMAQ Create"("Image Name"="untitled", "Image Type"=w813) -> ("New Image"=w810:T2)  [unwired: 3 in, 1 out]
      n173 = call <vilib>:"Application Directory.vi"() -> ("Application Directory"=w791:path)
      n174 = Build Path(base path=w791, name or relative path="_trap_screen_positions") -> (appended path=w799:path)
      n175 = Open/Create/Replace File(file path (use dialog)=w799, operation (0:open)=T25."open or create", access (0:read/write)=enum16{"read/write", "read-only", "write-only"}."read/write") -> (refnum out=w801:refnum<file>)  [unwired: 3 in, 2 out]
      n176 = local read "Trap Sets"() -> (w793:u32)
      n177 = for "Load trap positions on video screen from file." {
        N: w793 -> [_]
        tunnel: [w824] -> w794
        tunnel: w801 -> [w823]
        tunnel: [w820] -> w790 mode=indexing
        w822 = 4
        n178 = for {
          N: w822 -> [_]
          tunnel: [w828] -> w824
          tunnel: w823 -> [w827]
          tunnel: w822 -> [w826]
          tunnel: [w825] -> w821 mode=indexing
          n179 = Read from Binary File(5:w826, 11:w827) -> (2:w825:i32, 3:w828:refnum<file>)  [unwired: 4 in, 2 out]
        }
        n180 = Array To Cluster(array=w821) -> (cluster=w820:T29)
      }
      n181 = node-c288() -> (w819:T26)  [unwired: 4 in]
      n182 = timed-loop "acquire video and stage position" {
        timing: w819 -> [_]
        timing-out: [_] -> w818
        tunnel: w812 -> [w847]
        tunnel: w811 -> [w846]
        tunnel: w810 -> [w845]
        tunnel: [w844] -> w807
        tunnel: [w841] -> w806
        tunnel: [w842] -> w805
        tunnel: w804 -> [_]
        shift-right: [w838] -> w803
        shift-left: w790 -> [w839]
        tunnel: w793 -> [w836]
        stop <- w843 stop-if-true
        n183 = node-c288() -> ()  [unwired: 1 in, 1 out]
        n184 = event shown="[2] \"Primary Video Display\": Mouse Down" {
          selector: _ -> [_ _ _ _]
          dyn-events: _ -> [_ _ _ _]
          timeout: 10 -> [_ _ _ _]
          tunnel: w847 -> [w858 w873 w882 w901]
          tunnel: w846 -> [w857 w875 w880 w903]
          tunnel: w845 -> [w856 w874 w881 w902]
          tunnel: [w855 w873 w882 w901] -> w844
          tunnel: [w848 w877 FALSE FALSE] -> w843
          tunnel: [w852 w875 w880 w903] -> w842
          tunnel: [w851 w874 w881 w902] -> w841
          tunnel: "radius" -> [_ _ w887 _]
          tunnel: w839 -> [w849 w876 w885 _]
          tunnel: [w849 w876 w886 cluster{i32, i32, i32, i32}[] []] -> w838
          tunnel: w836 -> [_ _ w878 _]
          event Timeout {
            n185 = event-data() -> ()  [unwired: 1 in, 2 out]
            n186 = call <vilib>:"IMAQ Grab Acquire.vi"("error in (no error)"=w857, "Image In"=w856, "IMAQ Session In"=w858) -> ("error out"=w853:errorcluster, "Image Out"=w854:T2, "IMAQ Session Out"=w855:refnum<k11>)  [unwired: 5 in, 1 out]
            n187 = case shown="True" "trap\nmarkers?" {
              tunnel: w849 -> [_ w866]
              tunnel: w854 -> [w860 w865]
              tunnel: w853 -> [w859 w864]
              tunnel: [w859 w863] -> w852
              tunnel: [w860 w861] -> w851
              frame False {
              }
              frame True {
                n188 = for {
                  tunnel: w866 -> [w872] mode=indexing
                  shift-right: [w870] -> w861
                  shift-left: w865 -> [w871]
                  tunnel: w864 -> [w869]
                  tunnel: [w868] -> w863
                  tunnel: u32 16711680 ("Color") -> [w867]
                  n189 = call "IMAQ Overlay Oval"("Color"=w867, "error in (no error)"=w869, "Bounding Rectangle"=w872, "Image"=w871) -> ("error out"=w868:errorcluster, "Image Out"=w870:T2)  [unwired: 6 in]
                }
              }
            }
            "Primary Video Display" <- w851
            n190 = Unbundle By Name(w853) -> ("status"=w848:bool)
          }
          event "Stop All": Value Change {
            n191 = event-data() -> ()  [unwired: 1 in, 5 out]
            n192 = local read "Stop All"() -> (w877:bool)
          }
          event "Primary Video Display": Mouse Down {
            n193 = event-data() -> ()  [unwired: 1 in, 7 out]
            n194 = Array Size(array=w885) -> (size(s)=w884:i32)
            n195 = Less?(x=w884, y=w878) -> (x < y?=w883:bool)
            n196 = case shown="True" w883 {
              tunnel: w887 -> [_ w897]
              tunnel: w885 -> [w888 w891]
              tunnel: [w888 w890] -> w886
              frame False {
              }
              frame True {
                n197 = property on="Primary Video Display" class="ImageControl"() -> ("Last Mouse Position"=w889:cluster{"X":i32, "Y":i32})  [unwired: 2 in, 2 out]
                n198 = Unbundle By Name(w889) -> ("X"=w899:i32, "Y"=w898:i32)
                n199 = Add(x=w898, y=w897) -> (x+y=w895:i32)
                n200 = Subtract(x=w898, y=w897) -> (x-y=w893:i32)
                n201 = Add(x=w899, y=w897) -> (x+y=w894:i32)
                n202 = Subtract(x=w899, y=w897) -> (x-y=w896:i32)
                n203 = Bundle(w896, w895, w894, w893) -> (w892:cluster{i32, i32, i32, i32})  [unwired: 1 in]
                n204 = Build Array (concatenate)(w891, w892) -> (w890:T30)
              }
            }
          }
          event "clear markers": Value Change {
            n205 = event-data() -> ()  [unwired: 1 in, 5 out]
          }
        }
        n206 = node-c288() -> ()  [unwired: 1 in, 1 out]
      }
      n207 = node-c288(w818) -> ()  [unwired: 1 out]
      n208 = Set File Position(offset (in bytes) (0)=i64 0, refnum=w794, from (0:start)=enum16{"start", "end", "current"}."start") -> (refnum out=w795:refnum<file>)  [unwired: 1 in, 1 out]
      n209 = for "Write trap positions to file so they can be remembered\nwhen program is removed from memory" {
        tunnel: w803 -> [w832] mode=indexing
        tunnel: [w830] -> w802
        tunnel: w795 -> [w829]
        n210 = Cluster To Array(cluster=w832) -> (array=w831:i32[])
        n211 = for {
          tunnel: w831 -> [w835] mode=indexing
          tunnel: [w834] -> w830
          tunnel: w829 -> [w833]
          n212 = Write to Binary File(file (use dialog)=w833, data=w835) -> (refnum out=w834:refnum<file>)  [unwired: 4 in, 2 out]
        }
      }
      n213 = Close File(refnum=w802) -> ()  [unwired: 1 in, 2 out]
      n214 = call <vilib>:"IMAQ Stop.vi"("error in (no error)"=w805, "IMAQ Session In"=w807) -> ("error out"=w809:errorcluster, "IMAQ Session Out"=w808:refnum<k11>)  [unwired: 8 in]
      n215 = call "IMAQ Dispose"("Image"=w806) -> ()  [unwired: 5 in, 1 out]
      n216 = call <vilib>:"IMAQ Close.vi"("error in (no error)"=w809, "IMAQ Session In"=w808) -> ()  [unwired: 9 in, 1 out]
    }
    frame Enabled {
    }
  }
  n217 = call <vilib>:"Initialize Mouse.vi"() -> ("error out"=w20:errorcluster, "device ID"=w21:refnum<k1>)  [unwired: 10 in]
  n218 = node-c288() -> (w6:T26)  [unwired: 4 in]
  n219 = call-poly <vilib>:"Acquire Input Data.vi"("device ID"=w21, "error in (no error)"=w20) -> ("device ID"=w22:refnum<k1>, "error out"=w19:errorcluster)  [unwired: 14 in, 2 out]
  n220 = timed-loop {
    tunnel: w22 -> [w916]
    tunnel: [w915] -> w23
    tunnel: [w914] -> _
    tunnel: w19 -> [w913]
    tunnel: w18 -> [_]
    shift-right: ["Use mouse to move stage\n(press mouse wheel to quit)"] -> _
    shift-left: _ -> [w910]
    timing: w6 -> [_]
    timing-out: [_] -> w5
    i -> [w909]
    stop <- w912 stop-if-true
    n221 = node-c288() -> ()  [unwired: 1 in, 1 out]
    n222 = case shown="True" "Use mouse to move stage\n(press mouse wheel to quit)" {
      tunnel: w916 -> [w926 w946]
      tunnel: [w926 w968] -> w915
      tunnel: [w919 w950] -> w914
      tunnel: w913 -> [w920 w944]
      tunnel: w910 -> [_ w947]
      tunnel: w909 -> [_ w942]
      frame False {
        n223 = case shown="True" "reset motor comm. link" {
          tunnel: [w927 w930] -> w921
          tunnel: w920 -> [w927 w929]
          frame False {
          }
          frame True {
            n224 = call "CONEX_FUNCTIONAL_GLOBAL.vi"("error in"=w929, "Command"=T23."CLOSE") -> ("error out"=w932:errorcluster)  [unwired: 7 in, 2 out]
            n225 = flat-sequence {
              tunnel: w932 -> [w935]
              tunnel: [w935] -> w931
              frame #0 {
                n226 = Wait (ms)(milliseconds to wait=u32 50) -> ()  [unwired: 1 out]
              }
            }
            n227 = local write "reset motor comm. link"(FALSE ("reset motor comm. link")) -> ()
            n228 = call "CONEX_FUNCTIONAL_GLOBAL.vi"("error in"=w931, "Command"=T23."INIT") -> ("error out"=w930:errorcluster)  [unwired: 7 in, 2 out]
          }
        }
        n229 = call "CONEX_FUNCTIONAL_GLOBAL.vi"("Axis"=enum16{"X", "Y", "Z", "XY", "XZ", "YZ", "XYZ"}."XYZ", "error in"=w921, "Command"=T23."GET POS") -> ("error out"=w919:errorcluster, "Current Position"=w923:dbl[])  [unwired: 6 in, 1 out]
        n230 = local write "Current Position"(w923) -> ()
      }
      frame True {
        # "put cursor somewhere\nwhere mouse clicks and \nmouse wheel moves won't\nbe heard by the window"
        n231 = Not(x=w947) -> (.not. x?=w948:bool)
        n232 = Quotient & Remainder(x=w942, y=10) -> (x-y*floor(x/y)=w940:i32)  [unwired: 1 out]
        n233 = case shown="True" w948 {
          tunnel: w946 -> [w972 w976]
          tunnel: [w972 w975] -> w945
          tunnel: w944 -> [w971 w974]
          tunnel: [w971 w973] -> w943
          frame False {
          }
          frame True {
            n234 = call-poly <vilib>:"Acquire Input Data.vi"("device ID"=w976, "error in (no error)"=w974) -> ("device ID"=w975:refnum<k1>, "error out"=w973:errorcluster)  [unwired: 14 in, 2 out]
          }
        }
        n235 = Equal To 0?(x=w940) -> (x = 0?=w939:bool)
        n236 = case shown="True" w939 {
          frame False {
          }
          frame True {
            # "SetCursorPos"
            n237 = dll-call lib="User32.dll" fn="SetCursorPos"(900, 600) -> ()  [unwired: 5 in, 3 out]
          }
        }
        n238 = call-poly <vilib>:"Acquire Input Data.vi"("device ID"=w945, "key mode"=enum16{"RELATIVE", "ABSOLUTE"}."RELATIVE", "error in (no error)"=w943) -> ("device ID"=w968:refnum<k1>, "axis info"=w966:T31, "error out"=w949:errorcluster)  [unwired: 13 in, 1 out]
        n239 = Cluster To Array(cluster=w966) -> (array=w964:i32[])
        n240 = Compound Arithmetic op=MULTIPLY(invert 10000.0 ("value"), "mouse sensitivity", w964) -> (w962:dbl[])
        n241 = call "subVI_explode3array.vi"("Array"=w962) -> ("x"=w954:dbl, "y"=w953:dbl, "z"=w961:dbl)  [unwired: 12 in]
        n242 = case shown="False" "invert y?" {
          tunnel: w953 -> [w977 w979]
          tunnel: [w977 w978] -> w952
          frame False {
          }
          frame True {
            n243 = Negate(x=w979) -> (-x=w978:dbl)
          }
        }
        n244 = case shown="False" "invert x?" {
          tunnel: w954 -> [w980 w982]
          tunnel: [w980 w981] -> w951
          frame False {
          }
          frame True {
            n245 = Negate(x=w982) -> (-x=w981:dbl)
          }
        }
        n246 = Reciprocal(x="Z sensitivity") -> (1/x=w937:dbl)
        n247 = Divide(x=w961, y=w937) -> (x/y=w960:dbl)
        n248 = Build Array(w951, w952, w960) -> (w957:dbl[])
        n249 = call "CONEX_FUNCTIONAL_GLOBAL.vi"("Axis"=enum16{"X", "Y", "Z", "XY", "XZ", "YZ", "XYZ"}."XYZ", "error in"=w949, "Position"=w957, "Command"=T23."REL MOVE") -> ("error out"=w950:errorcluster)  [unwired: 5 in, 2 out]
      }
    }
    n250 = local read "Stop All"() -> (w912:bool)
    n251 = node-c288() -> ()  [unwired: 1 in, 1 out]
  }
  n252 = node-c288(i64 1 ("Period"), 1 ("Processor")) -> (w169:T26)  [unwired: 2 out]
  n253 = node-c288(2 ("Processor")) -> (w9:T26)  [unwired: 3 in]
  n254 = node-c288() -> (w74:T26)  [unwired: 4 in]
  n255 = node-c288() -> (w81:T26)  [unwired: 4 out]
  n256 = timed-loop "Acquire Data" {
    tunnel: w18 -> [w1239]
    tunnel: w41 -> [w1238]
    tunnel: [w1269] -> w32
    tunnel: [w1263] -> w31
    timing: w169 -> [_]
    timing-out: [_] -> w168
    tunnel: w64 -> [w1069]
    stop <- "Stop All" stop-if-true
    (unwired) u32 0 ("Number of Elements")
    w1056 = "NI_ChannelName" ("name")
    n257 = node-c288() -> ()  [unwired: 2 out]
    n258 = First Call?() -> (First Call?: T/F=w1022:bool)
    n259 = Or(x="Reset", y=w1022) -> (x .or. y?=w1023:bool)
    n260 = case "Reset data stream" shown="True" w1023 {
      tunnel: w1239 -> [w1355 w1363]
      tunnel: w1238 -> [w1354 w1362]
      tunnel: [w1355 w1357] -> w1234
      tunnel: [w1354 w1356] -> w1233
      frame False {
      }
      frame True {
        w1360 = TRUE ("AI to FIFO")
        n261 = local write "Overflow (data lost)"(FALSE ("Overflow (data lost)")) -> ()
        n262 = call "reset FPGA DMA.vi"("error in"=w1362, "FPGA VI Reference In"=w1363) -> ("error out"=w1358:errorcluster, "FPGA VI Reference Out"=w1359:T20)
        n263 = xnode "Read/Write Control"("FPGA VI Reference In"=w1359, "error in"=w1358, "AI to FIFO"=w1360, "APD to FIFO"=w1360) -> ("FPGA VI Reference Out"=w1357:T20, "error out"=w1356:errorcluster)
      }
    }
    n264 = Or(x="Start AOD Scan", y="Trap Raster Scan") -> (x .or. y?=w1186:bool)
    n265 = case "Start AOM raster scan" shown="False" w1186 {
      tunnel: w1234 -> [w2963 w2973]
      tunnel: w1233 -> [w2962 w2972]
      tunnel: [w2963 w2966] -> w1232
      tunnel: [w2962 w2965] -> w1231
      frame False {
      }
      frame True {
        n266 = case shown="True" "Restart DMA? (AOD)" {
          tunnel: [w3384 w3386] -> w2967
          tunnel: [w3383 w3385] -> w2968
          tunnel: w2973 -> [w3384 w3388]
          tunnel: w2972 -> [w3383 w3387]
          frame False {
          }
          frame True {
            n267 = local write "Overflow (data lost)"(FALSE ("Overflow (data lost)")) -> ()
            n268 = call "reset FPGA DMA.vi"("error in"=w3387, "FPGA VI Reference In"=w3388) -> ("error out"=w3385:errorcluster, "FPGA VI Reference Out"=w3386:T20)
          }
        }
        n269 = local write "Trap Raster Scan"(FALSE ("Trap Raster Scan")) -> ()
        n270 = case shown="True" "Move MCL Also?" {
          tunnel: w2968 -> [w2976 w3085]
          tunnel: w2967 -> [w2977 w3086]
          tunnel: [w2975 w3089] -> w2966
          tunnel: [w2974 w3088] -> w2965
          frame False {
            w2978 = TRUE ("AI to FIFO")
            n271 = xnode "Read/Write Control"("FPGA VI Reference In"=w2977, "error in"=w2976, "AI to FIFO"=w2978, "APD to FIFO"=w2978, "Start scan"=w2978) -> ("FPGA VI Reference Out"=w2975:T20, "error out"=w2974:errorcluster)
          }
          frame True {
            w3082 = FALSE ("1D or 2D Scan?")
            w3087 = TRUE ("AI to FIFO")
            # "Count for MCL loop"
            # "N total cycles"
            # "N steps"
            # "V_int"
            n272 = local read "Scan Range (nm)"() -> (w3064:dbl)
            n273 = local read "Number of F/B Scans (AOD)"() -> (w3081:u16)
            n274 = Sign(1:w3064) -> (0:w3063:dbl)
            n275 = Compound Arithmetic op=MULTIPLY(w3064, "MCL Step Position Ratio", "MCL/AOM Scale Tweak") -> (w3068:dbl)
            n276 = Negate(x=w3063) -> (-x=w3060:dbl)
            n277 = Multiply(x=w3060, y="MCL Step Increment (V_int)") -> (x*y=w3062:dbl)
            n278 = Divide(x=w3068, y="MCL X Cal (nm/V)") -> (x/y=w3074:dbl)
            n279 = Multiply(x=32767.0 ("y"), y=w3074) -> (x*y=w3080:dbl)
            n280 = local read "Total Counts (ticks)"() -> (w3065:u32)
            n281 = local read "Cycles/step (AOD)"() -> (w3076:u64)
            n282 = local read "Scan steps (AOD)"() -> (w3077:u64)
            n283 = Divide(x=w3080, y=10.0) -> (x/y=w3073:dbl)
            n284 = Divide(x=w3073, y="MCL Step Increment (V_int)") -> (x/y=w3071:dbl)
            n285 = Absolute Value(x=w3071) -> (abs(x)=w3059:dbl)
            n286 = Compound Arithmetic op=MULTIPLY(w3077, w3076, w3065) -> (w3072:u64)
            n287 = local write "wait to reset values"(w3087) -> ()
            n288 = local write "MCL Scanning"(w3087) -> ()
            n289 = Divide(x=w3072, y=w3059) -> (x/y=w3069:dbl)
            "MCL Count" <- w3069
            n290 = xnode "Read/Write Control"("FPGA VI Reference In"=w3086, "error in"=w3085, "Scan steps (MCL)"=w3059, "Number of scans (MCL)"=w3081, "Cycles per step (MCL)"=u64 1, "Scan freq.  increment (MCL)"=w3062, "1D or 2D Scan?"=w3082, "MCL Scan Axis"=w3082, "Cont. Scan (MCL)"=w3082, "MCL count"=w3069) -> ("FPGA VI Reference Out"=w3084:T20, "error out"=w3083:errorcluster)